vi "crop.vi"(0 "Particle Measurements (Pixels)":dbl[][](array[numeric]) format="%.2f", 1 "Number of Particles":i32, 2 "cropWidth":i32=1200, 3 "cropped Image":T1, 4 "std threshold":sgl, 5 "raw image":T1=refnum, 9 "processed image":T1=refnum, 10 "downsampling":i32, 11 "Standard Variation":sgl, 12 "buffer number":u32, 13 "cropHeight":i32=600, 14 "error in":errorcluster) -> (6 "error out":errorcluster, 8 "raw image out":T1, 15 "cropped image out":T1)   [LabVIEW 2012]
uses:
  <vilib>/vision/Image Controls.llb/IMAQ Image.ctl
  GlobalBaslerCamera.vi
  <vilib>/imath/engines/lvmath2/RunTimeEngine/ErrorHandling/NIMS_Finalize Error.vi
  <vilib>/imath/engines/lvmath2/RunTimeEngine/NodeEndStatement/NIMS_NodeEndStatement_Output.vi
  <instcachedir>/0/NIMS_NodeEndStatement_Output_53EC0D466D134D7ABD903AC30B43404B.lvgen/NIMS_NodeEndStatement_Output_53EC0D466D134D7ABD903AC30B43404B_004.vi
  <vilib>/imath/engines/lvmath2/RunTimeEngine/RangeToken/NIMS_Range_R2.vi
  <vilib>/imath/engines/lvmath2/RunTimeEngine/VariableToken/Read/NIMS_Get Elements - SorM(_) - Check.vi
  <instcachedir>/0/NIMS_Get Elements - SorM(_) - Check_8FDA2664A675493882C25203DD903B51.lvgen/NIMS_Get Elements - SorM(_) - Check_8FDA2664A675493882C25203DD903B51_001.vi
  <vilib>/imath/engines/lvmath2/RunTimeEngine/BuiltInFunctions/round/NIMS_round(DBL-M).vi
  <vilib>/imathl/engines/lvmath/Functions/Error Handling/Create Error.vi
  <instcachedir>/0/NIMS_Get Elements - SorM(_) - Check_8FDA2664A675493882C25203DD903B51.lvgen/NIMS_Get Elements - SorM(_) - Check_8FDA2664A675493882C25203DD903B51_000.vi
  <vilib>/imath/engines/lvmath2/RunTimeEngine/ReplaceToken/NIMS_Replace - Check Linear.vi
  <instcachedir>/0/NIMS_Replace - Check Linear_44ABB4D6A819426DBDF25CCE6827BF1D.lvgen/NIMS_Replace - Check Linear_44ABB4D6A819426DBDF25CCE6827BF1D_001.vi
  <vilib>/imath/engines/lvmath2/RunTimeEngine/ReplaceToken/NIMS_Replace - Size Check _(_)=S.vi
  <instcachedir>/0/NIMS_Replace - Size Check _(_)=S_5AC8AA27B9694BB9828B57BCF666F597.lvgen/NIMS_Replace - Size Check _(_)=S_5AC8AA27B9694BB9828B57BCF666F597_000.vi
  <vilib>/imath/engines/lvmath2/RunTimeEngine/ReplaceToken/NIMS_Replace - V(S)=S.vi
  <instcachedir>/0/NIMS_Replace - V(S)=S_927EF1B21AA84780A9A306EC96B904EC.lvgen/NIMS_Replace - V(S)=S_927EF1B21AA84780A9A306EC96B904EC_000.vi
  <vilib>/imath/engines/lvmath2/RunTimeEngine/ErrorHandling/NIMS_Create Error From Enums.vi
  <instcachedir>/0/NIMS_Replace - Check Linear_44ABB4D6A819426DBDF25CCE6827BF1D.lvgen/NIMS_Replace - Check Linear_44ABB4D6A819426DBDF25CCE6827BF1D_008.vi
  <instcachedir>/0/NIMS_Replace - Size Check _(_)=S_5AC8AA27B9694BB9828B57BCF666F597.lvgen/NIMS_Replace - Size Check _(_)=S_5AC8AA27B9694BB9828B57BCF666F597_007.vi
  <instcachedir>/0/NIMS_Replace - V(S)=S_927EF1B21AA84780A9A306EC96B904EC.lvgen/NIMS_Replace - V(S)=S_927EF1B21AA84780A9A306EC96B904EC_003.vi
  daq test/GlobalStatus.vi
  <vilib>/vision/NI_Vision_Development_Module.lvlib
  <resource>/objmgr/IMAQImage.rc
panel:
  out "Image Size":cluster{"x":i32, "y":i32}
  out "out of focus":bool
  out "saving to disk":bool
  out "touching borders":bool
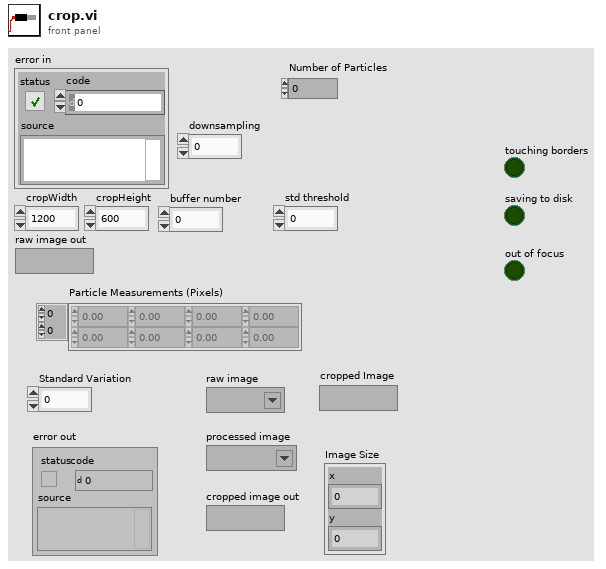
[diagram p1: front panel]
types:
  T1 = typedef "IMAQ Image.ctl" = refnum<image>
  T2 = typedef "Semaphore RefNum" = refnum<k1>
  T3 = cluster{"rectangle[0]":i32, "rectangle[1]":i32, "rectangle[2]":i32, "rectangle[3]":i32}
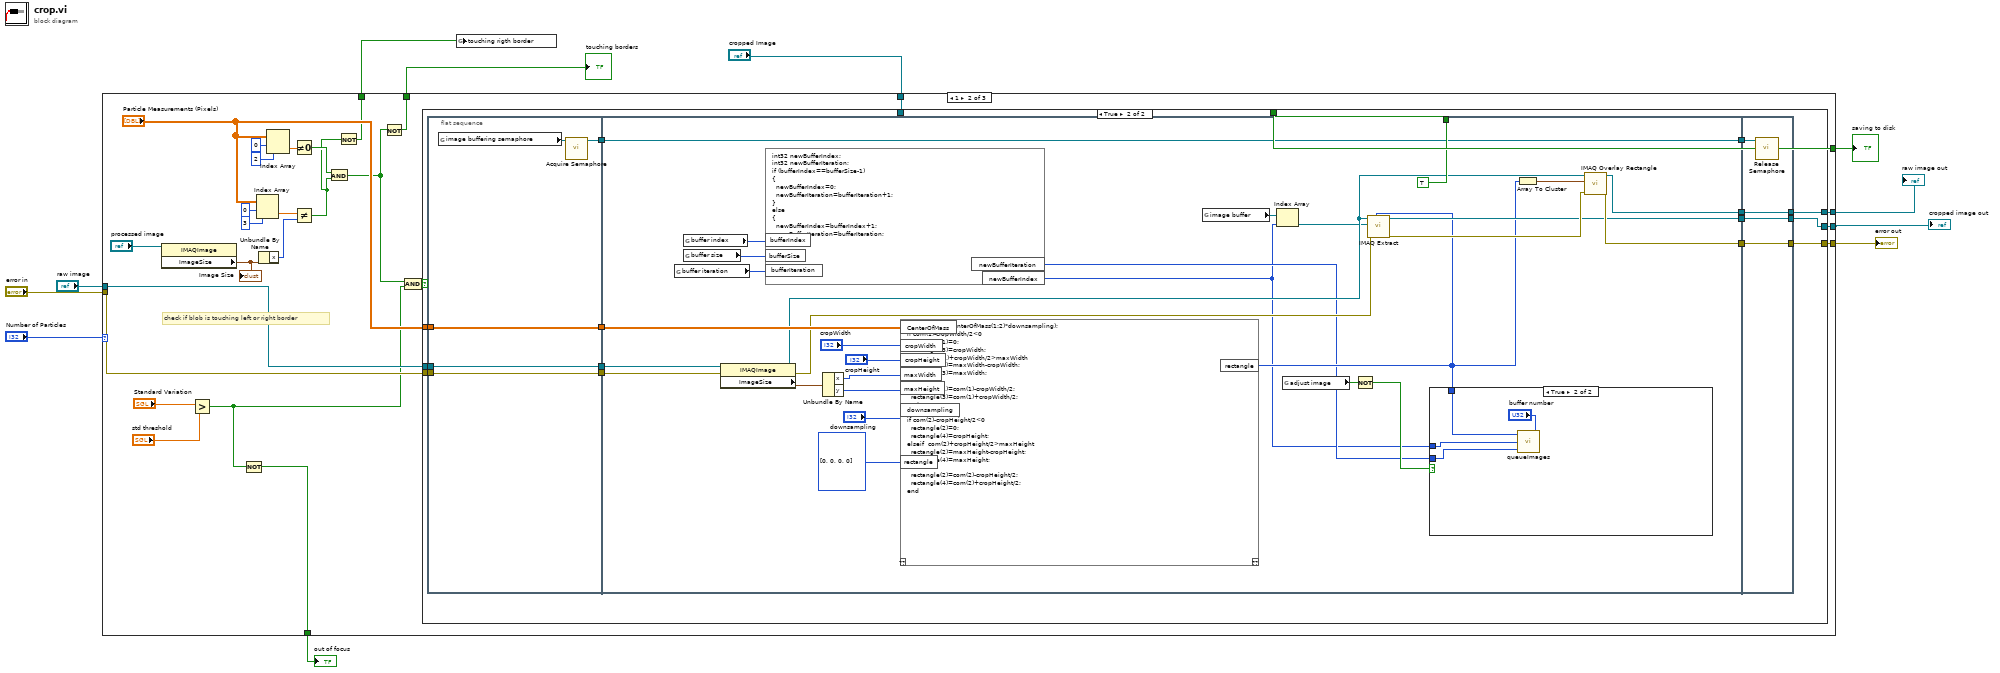
[diagram p0: block diagram]
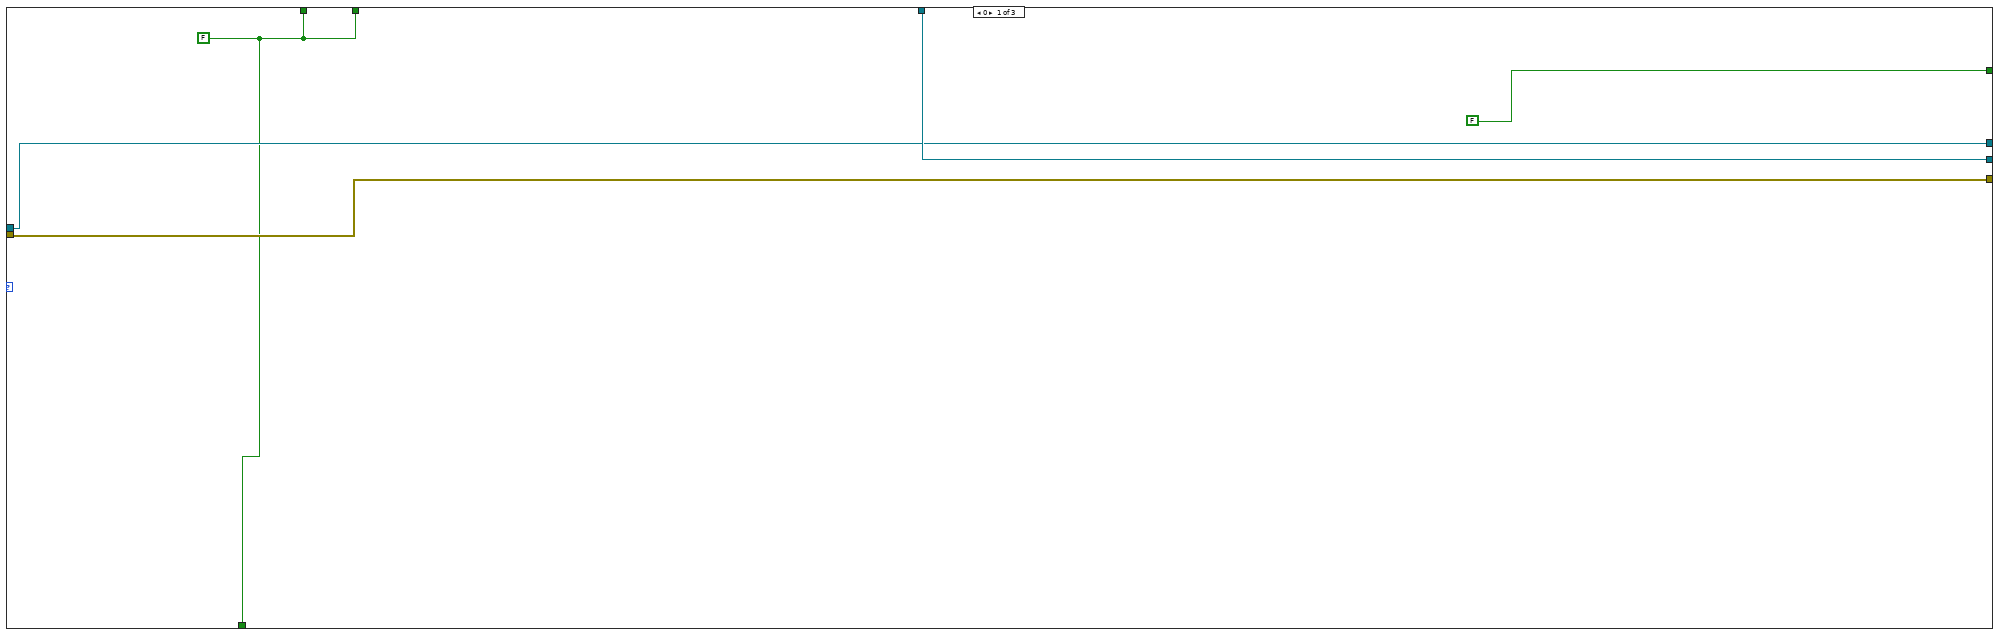
[diagram p2: hidden frame]
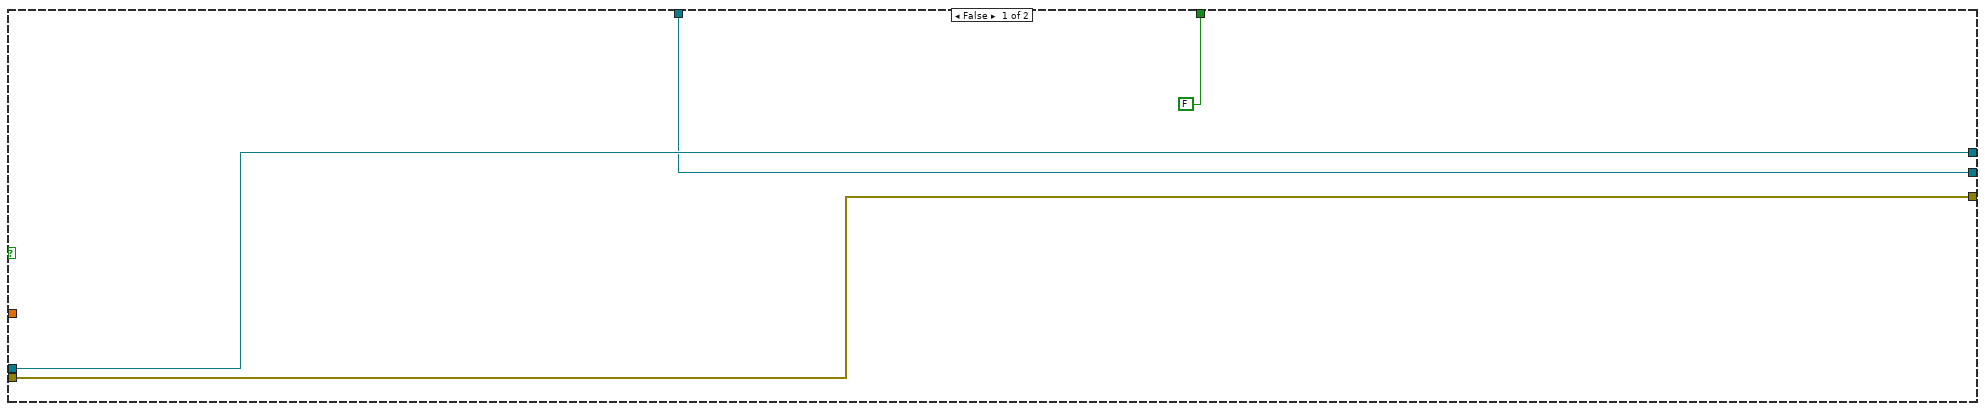
[diagram p3: hidden frame]
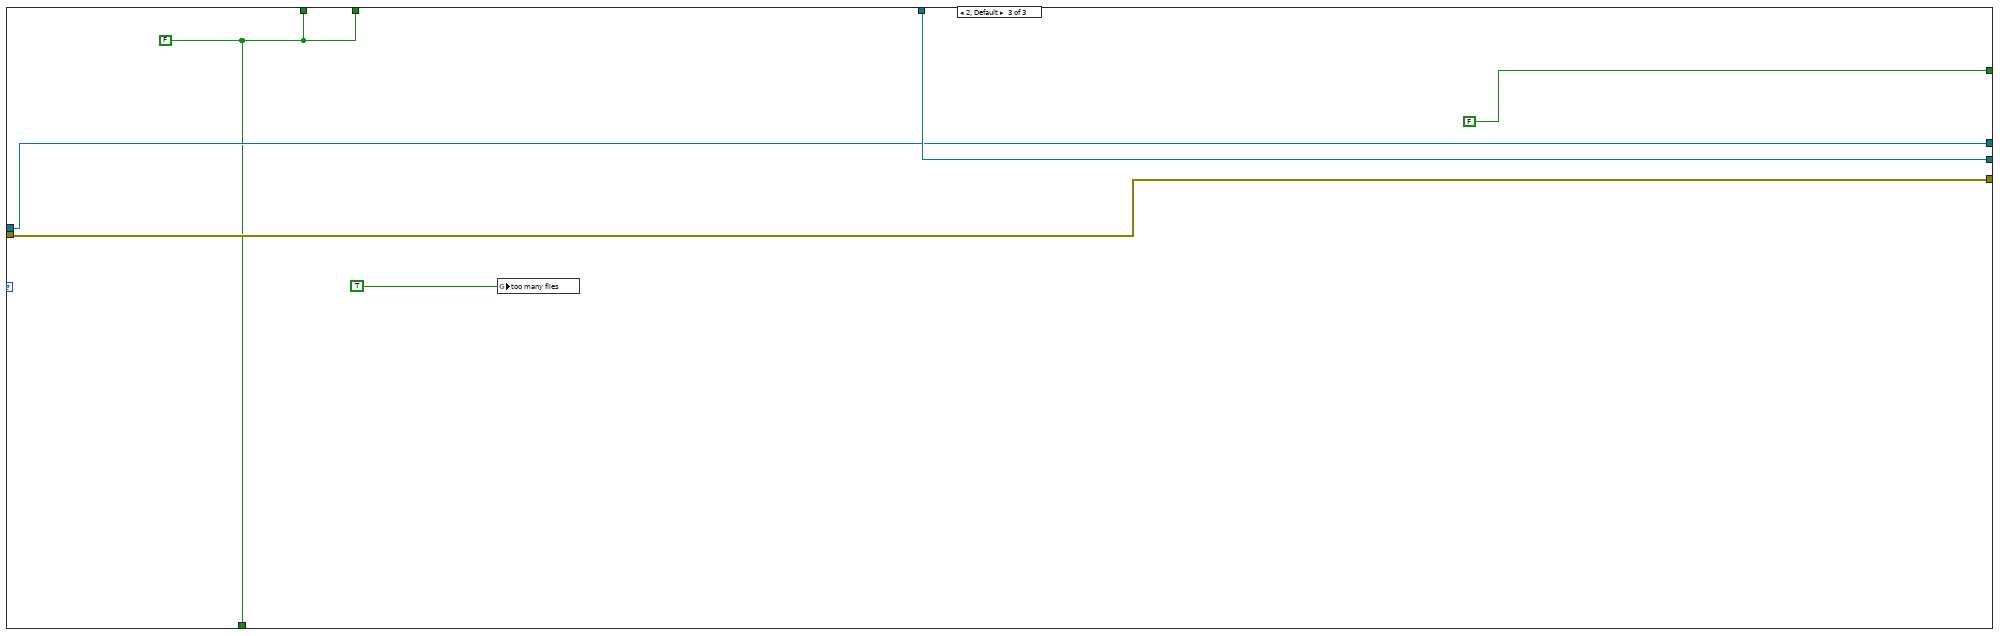
[diagram p5: hidden frame]
diagram:
  n1 = case shown="1" "Number of Particles" {
    tunnel: "error in" -> [w16 w33 w516]
    tunnel: "raw image" -> [w13 w34 w512]
    tunnel: [w16 w43 w516] -> w9
    tunnel: [FALSE w32 FALSE] -> w7
    tunnel: [w12 w29 w511] -> w6
    tunnel: [w12 w27 w511] -> w5
    tunnel: [w14 w19 w513] -> w2
    tunnel: "cropped Image" -> [w14 w21 w513]
    tunnel: [w13 w20 w512] -> w3
    tunnel: [w12 w17 w511] -> w1
    frame 0 {
      w12 = FALSE
    }
    frame 1 {
      # "check if blob is touching left or right border"
      n2 = property class="IMAQImage"(reference="processed image") -> ("ImageSize"=w35:cluster{"x":i32, "y":i32})  [unwired: 1 in, 2 out]
      "Image Size" <- w35
      n3 = Greater?(x="Standard Variation", y="std threshold") -> (0:w26:bool)
      n4 = Not(x=w26) -> (.not. x?=w27:bool)
      n5 = Index Array(array="Particle Measurements (Pixels)", index (row)=0, index (col)=3 ("disabled index (col)")) -> (element=w25:dbl)
      n6 = Unbundle By Name(w35) -> ("x"=w24:i32)
      n7 = Index Array(array="Particle Measurements (Pixels)", index (row)=0, index (col)=2 ("disabled index (col)")) -> (element=w41:dbl)
      n8 = Not Equal To 0?(x=w41) -> (x != 0?=w23:bool)
      n9 = Not Equal?(x=w25, y=w24) -> (x != y?=w18:bool)
      n10 = And(x=w23, y=w18) -> (x .and. y?=w22:bool)
      n11 = Not(x=w18) -> (.not. x?=w17:bool)
      n12 = Not(x=w22) -> (.not. x?=w29:bool)
      n13 = And(x=w22, y=w26) -> (x .and. y?=w28:bool)
      n14 = case shown="True" w28 {
        tunnel: w34 -> [w45 w61]
        tunnel: [w47 w57] -> w43
        tunnel: "Particle Measurements (Pixels)" -> [_ w62]
        tunnel: w33 -> [w47 w60]
        tunnel: [FALSE w59] -> w32
        tunnel: w21 -> [w44 _]
        tunnel: [w45 w58] -> w20
        tunnel: [w44 w48] -> w19
        frame False {
        }
        frame True {
          n15 = flat-sequence {
            tunnel: w60 -> [w65]
            tunnel: w61 -> [w66]
            tunnel: w62 -> [w67]
            tunnel: [w67] -> w56
            tunnel: [w66] -> w55
            tunnel: [w65] -> w54
            tunnel: [w63] -> w53
            tunnel: [TRUE] -> w59
            tunnel: w56 -> [w93]
            tunnel: w55 -> [w88]
            tunnel: w54 -> [w87]
            tunnel: w53 -> [w68]
            tunnel: [w82] -> w52
            tunnel: [w80] -> w51
            tunnel: [w79] -> w50
            tunnel: [w68] -> w49
            tunnel: [w508] -> w48
            tunnel: [w509] -> w57
            tunnel: [w510] -> w58
            tunnel: w52 -> [w510]
            tunnel: w51 -> [w509]
            tunnel: w50 -> [w508]
            tunnel: w49 -> [w507]
            frame #0 {
              n16 = global read "GlobalBaslerCamera.vi" "image buffering semaphore"() -> (w64:T2)
              n17 = call <vilib>:"Acquire Semaphore.vi"("semaphore"=w64) -> ("semaphore out"=w63:T2)  [unwired: 4 in, 2 out]
            }
            frame #1 {
              n18 = global read "GlobalBaslerCamera.vi" "buffer iteration"() -> (w74:i32)
              n19 = global read "GlobalBaslerCamera.vi" "buffer index"() -> (w75:i32)
              n20 = global read "GlobalBaslerCamera.vi" "buffer size"() -> (w76:i32)
              n21 = property class="IMAQImage"(reference=w88, error in=w87) -> (reference out=w83:T1, error out=w89:errorcluster, "ImageSize"=w91:cluster{"x":i32, "y":i32})
              n22 = formula code="int32 newBufferIndex;\nint32 newBufferIteration;\nif (bufferIndex==bufferSize-1)\n{\n  newBufferIndex=0;\n  newBufferIteration=bufferIteration+1;\n}\nelse\n{\n  newBufferIndex=bufferIndex+1;\n  newBufferIteration=bufferIteration;\n}"("bufferIndex"=w75, "bufferSize"=w76, "bufferIteration"=w74) -> ("newBufferIndex"=w69:i32, "newBufferIteration"=w70:i32)
              n23 = Unbundle By Name(w91) -> ("x"=w92:i32, "y"=w90:i32)
              n24 = mathscript code="com = round(CenterOfMass(1:2)*downsampling);\nif com(1)-cropWidth/2<0\n  rectangle(1)=0;\n  rectangle(3)=cropWidth;\nelseif  com(1)+cropWidth/2>maxWidth\n  rectangle(1)=maxWidth-cropWidth;\n  rectangle(3)=maxWidth;\nelse\n  rectangle(1)=com(1)-cropWidth/2;\n  rectangle(3)=com(1)+cropWidth/2;\nend\n\nif com(2)-cropHeight/2<0\n  rectangle(2)=0;\n  rectangle(4)=cropHeight;\nelseif  com(2)+cropHeight/2>maxHeight\n  rectangle(2)=maxHeight-cropHeight;\n  rectangle(4)=maxHeight;\nelse\n  rectangle(2)=com(2)-cropHeight/2;\n  rectangle(4)=com(2)+cropHeight/2;\nend"("CenterOfMass"=w93, "cropWidth"="cropWidth", "maxWidth"=w92, "maxHeight"=w90, "cropHeight"="cropHeight", "downsampling"="downsampling", "rectangle"=i32[] [0, 0, 0, 0]) -> ("rectangle"=w72:i32[])  [unwired: 1 in, 1 out]
              n25 = global read "GlobalBaslerCamera.vi" "image buffer"() -> (w73:T1[])
              n26 = Index Array(array=w73, index=w69) -> (element=w71:T1)
              n27 = global read "GlobalBaslerCamera.vi" "adjust image"() -> (w78:bool)
              n28 = Not(x=w78) -> (.not. x?=w77:bool)
              n29 = call "IMAQ Extract"("Optional Rectangle"=w72, "error in (no error)"=w89, "Image Dst"=w71, "Image Src"=w83) -> ("error out"=w81:errorcluster, "Image Dst Out"=w79:T1)  [unwired: 6 in]
              n30 = case shown="True" w77 {
                tunnel: w72 -> [_ w100]
                tunnel: w70 -> [_ w97]
                tunnel: w69 -> [_ w98]
                frame False {
                }
                frame True {
                  n31 = call "queueImages.vi"("buffer number"="buffer number", "buffer iteration"=w97, "buffer index"=w98, "rectangle"=w100) -> ()
                }
              }
              n32 = Array To Cluster(array=w72) -> (cluster=w84:T3)
              n33 = call "IMAQ Overlay Rectangle"("error in (no error)"=w81, "Rectangle"=w84, "Image"=w83) -> ("error out"=w80:errorcluster, "Image Out"=w82:T1)  [unwired: 7 in]
            }
            frame #2 {
              n34 = call <vilib>:"Release Semaphore.vi"("semaphore"=w507) -> ()  [unwired: 5 in, 2 out]
            }
          }
        }
      }
    }
    frame 2, Default {
      w511 = FALSE
      n35 = global write "GlobalStatus.vi" "too many flies"(TRUE ("too many flies")) -> ()
    }
  }
  "error out" <- w9
  "touching borders" <- w6
  "saving to disk" <- w7
  "out of focus" <- w5
  "cropped image out" <- w2
  "raw image out" <- w3
  n36 = global write "GlobalBaslerCamera.vi" "touching rigth border"(w1) -> ()
